vi "for testing.vi"() -> ()   [LabVIEW 2016] (continued)
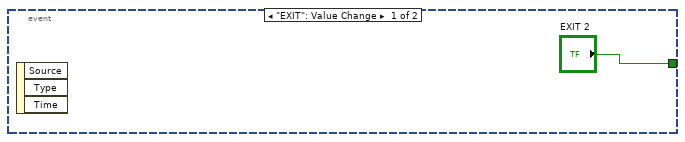
[diagram p2: hidden frame]
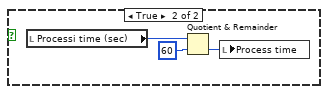
[diagram p3: hidden frame]
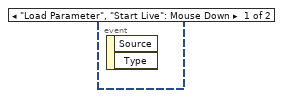
[diagram p4: hidden frame]
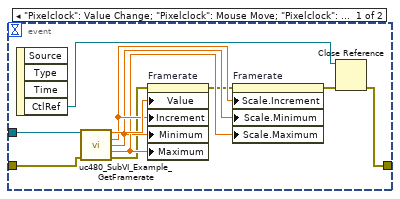
[diagram p5: hidden frame]
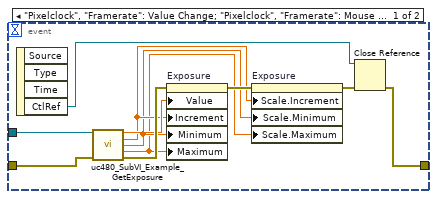
[diagram p6: hidden frame]
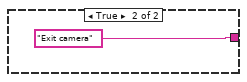
[diagram p7: hidden frame]
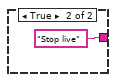
[diagram p8: hidden frame]
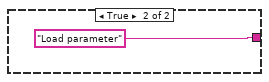
[diagram p9: hidden frame]
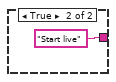
[diagram p10: hidden frame]
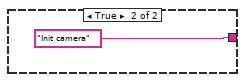
[diagram p11: hidden frame]
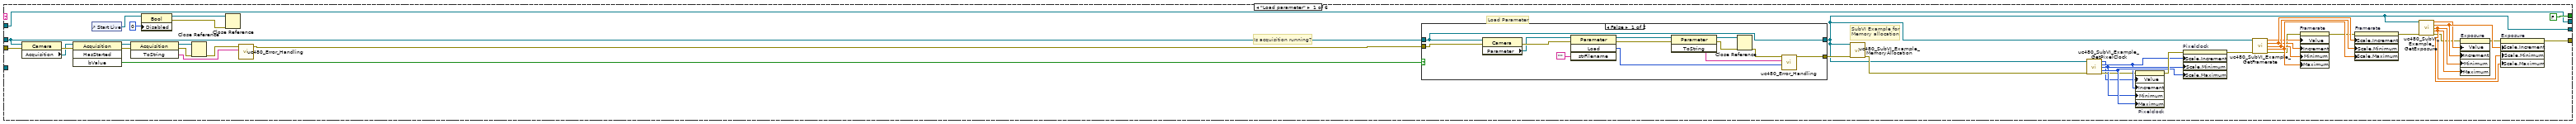
[diagram p12: hidden frame]
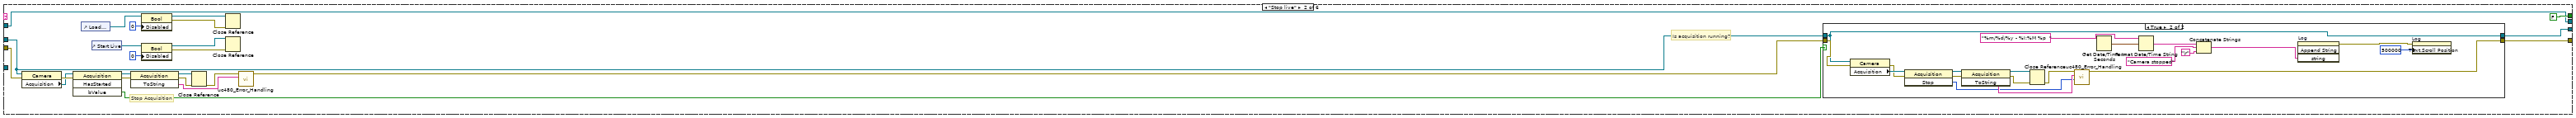
[diagram p14: hidden frame]
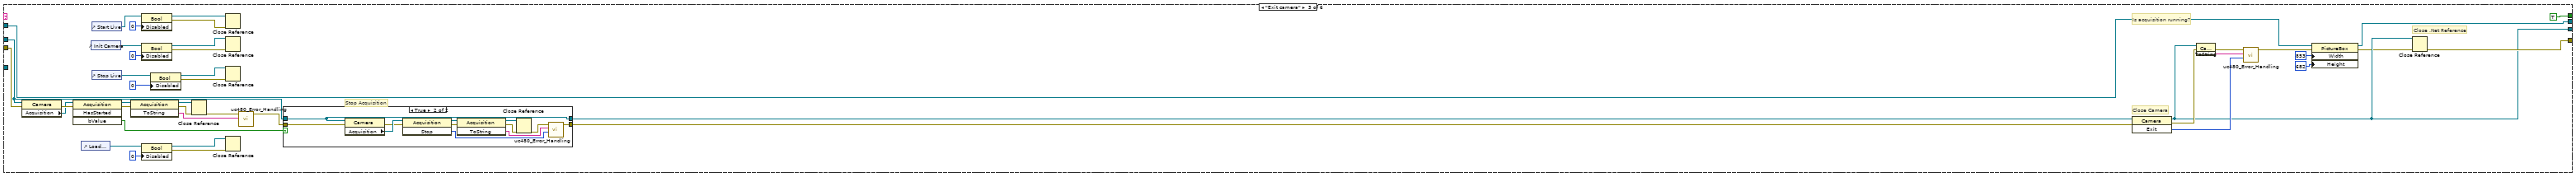
[diagram p16: hidden frame]
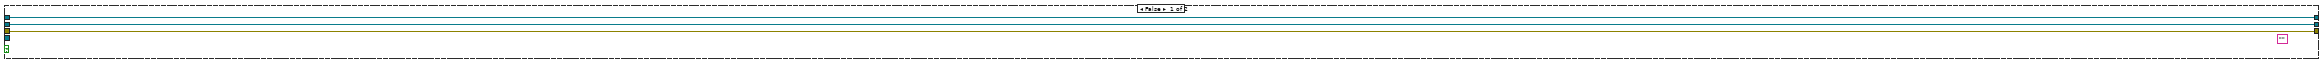
[diagram p18: hidden frame]
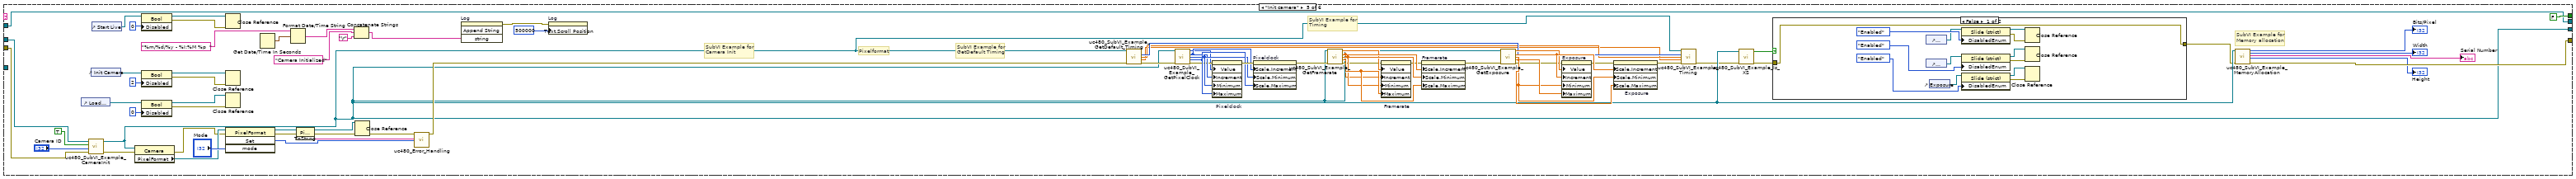
[diagram p20: hidden frame]
          }
          frame True {
            n522 = call "IR_Alignment_Diode.vi"("AD Action"=enum16{"AD Off", "AD On"}."AD On") -> ()  [unwired: 14 in, 1 out]
          }
        }
      }
      event "Open \nManual": Value Change {
        n523 = event-data() -> ()  [unwired: 1 in, 6 out]
        n524 = case shown="True" "Open \nManual" {
          tunnel: [_ "Opening Manual" ("StringOut")] -> w955
          frame False {
          }
          frame True {
            w962 = FALSE  # wait until completion? (T)
            n525 = control-ref of="This VI"() -> (w966:refnum<vi>)
            n526 = property class="VI"(reference=w966) -> ("Path"=w965:path)  [unwired: 1 in, 2 out]
            n527 = Strip Path(path=w965) -> (stripped path=w964:path)  [unwired: 1 out]
            n528 = Build Path(base path=w964, name or relative path="LAST_Software_Manual.PDF") -> (appended path=w958:path)
            n529 = Path To String(path=w958) -> (string=w959:string)
            n530 = Concatenate Strings("cmd  /c \"", w959, "\"" ("string")) -> (w956:string)
            n531 = call <vilib>:"System Exec.vi"("run minimized? (F)"=TRUE, "wait until completion? (T)"=w962, "command line"=w956) -> ()  [unwired: 5 in, 4 out]
          }
        }
      }
      event "Stages status": Value Change {
        w974 = "Ready"
        n532 = event-data() -> ()  [unwired: 1 in, 6 out]
        n533 = case shown="True" "Stages status" {
          tunnel: w983 -> [_ w996]
          tunnel: w982 -> [_ w995]
          tunnel: w981 -> [_ w994]
          tunnel: [w987 w993] -> w980
          tunnel: [w987 w991] -> w970
          tunnel: [w987 w992] -> w969
          frame False {
            w987 = ""
          }
          frame True {
            n534 = call <userlib>:"Open TCP-IP.vi"("IP address"=w996) -> ("error out"=w990:errorcluster, "Connection ID"=w997:T6)  [unwired: 8 in, 1 out]
            n535 = call <vilib>:"Simple Error Handler.vi"("error in (no error)"=w990) -> ("error?"=w988:bool, "error out"=w989:errorcluster)  [unwired: 4 in, 3 out]
            n536 = case shown="True" w988 {
              tunnel: w997 -> [w1018 _]
              tunnel: w989 -> [w1017 _]
              tunnel: w995 -> [w1010 _]
              tunnel: w994 -> [w1009 _]
              tunnel: [w1008 w1019] -> w993
              tunnel: [w1005 w1019] -> w992
              tunnel: [w1001 w1019] -> w991
              frame False {
                n537 = call "Get Stages Status.vi"("error in (no error)"=w1017, "Group Name (250 c max)"=w1010, "connection ID in"=w1018) -> ("error out"=w1014:errorcluster, "XPS error out"=w1013:errorcluster, "Group Status String"=w1005:string, "connection ID out"=w1016:T6)  [unwired: 4 in, 1 out]
                n538 = call "Get Stages Status.vi"("error in (no error)"=w1014, "XPS error in (no error)"=w1013, "Group Name (250 c max)"=w1009, "connection ID in"=w1016) -> ("error out"=w1011:errorcluster, "XPS error out"=w1007:errorcluster, "Group Status String"=w1001:string, "connection ID out"=w1012:T6)  [unwired: 3 in, 1 out]
                n539 = call <vilib>:"Simple Error Handler.vi"("error source (\" \")"="Stage status" ("error source (\" \")"), "error in (no error)"=w1007) -> ()  [unwired: 3 in, 5 out]
                n540 = Concatenate Strings("Axis 1 " ("string"), w1005) -> (w1004:string)
                n541 = call <userlib>:"Close TCP-IP.vi"("error in (no error)"=w1011, "connection ID in"=w1012) -> ("Error out"=w1006:errorcluster)  [unwired: 9 in]
                n542 = call <vilib>:"Simple Error Handler.vi"("error source (\" \")"="TCP close Stage status" ("error source (\" \")"), "error in (no error)"=w1006) -> ()  [unwired: 3 in, 5 out]
                n543 = Concatenate Strings("Axis 2 " ("string"), w1001) -> (w1002:string)
                n544 = Concatenate Strings(w1004, " - " ("string"), w1002) -> (w1008:string)
              }
              frame True {
                w1019 = ""
              }
            }
          }
        }
        n545 = String Subset(string=w969, offset (0)=0, length (rest)=5 ("length (rest)")) -> (substring=w973:string)
        n546 = String Subset(string=w970, offset (0)=0, length (rest)=5 ("length (rest)")) -> (substring=w975:string)
        n547 = Equal?(x=w974, y=w973) -> (x = y?=w971:bool)
        n548 = Equal?(x=w975, y=w974) -> (x = y?=w972:bool)
        n549 = And(x=w972, y=w971) -> (x .and. y?=w968:bool)
        n550 = case shown="True" w968 {
          frame False {
          }
          frame True {
            n551 = property on="Home Axes" class="Bool"("Visible"=TRUE) -> ()  [unwired: 2 in, 2 out]
            n552 = property on="Axes Manual Control" class="Bool (strict)"("Visible"=TRUE) -> ()  [unwired: 2 in, 2 out]
          }
        }
      }
      event "Save configuration": Value Change {
        n553 = event-data() -> ()  [unwired: 1 in, 6 out]
        n554 = case shown="True" "Save configuration" {
          frame False {
          }
          frame True {
            w1047 = "ROI Processing" ("section")
            n555 = control-ref of="This VI"() -> (w1053:refnum<vi>)
            n556 = property class="VI"(reference=w1053) -> ("Path"=w1052:path)  [unwired: 1 in, 2 out]
            n557 = Strip Path(path=w1052) -> (stripped path=w1051:path)  [unwired: 1 out]
            n558 = Build Path(base path=w1051, name or relative path="General_Configuration.ini") -> (appended path=w1049:path)
            n559 = local read "Heigth (µm)"() -> (w1033:i32)
            n560 = local read "Width (µm)"() -> (w1034:i32)
            n561 = local read "Pixel size"() -> (w1045:dbl)
            n562 = local read "X offset"() -> (w1032:i32)
            n563 = local read "Y offset"() -> (w1031:i32)
            n564 = local read "Height  step \ndivider"() -> (w1044:i32)
            n565 = call <vilib>:"Open Config Data.vi"("create file if necessary (T)"=FALSE, "configuration file path"=w1049) -> ("refnum"=w1021:T5)  [unwired: 7 in, 2 out]
            n566 = local read "Speed (µm/s)"() -> (w1035:i32)
            n567 = local read "Precision (%)"() -> (w1036:dbl)
            n568 = call-poly <vilib>:"Write Key.vi"("section"=w1047, "value"=w1045, "key"="Pixel Size", "refnum"=w1021) -> ("error out"=w1030:errorcluster)  [unwired: 5 in, 2 out]
            n569 = call-poly <vilib>:"Write Key.vi"("section"=w1047, "value"=w1044, "key"="Heigth step divider", "refnum"=w1021) -> ("error out"=w1029:errorcluster)  [unwired: 5 in, 2 out]
            n570 = call-poly <vilib>:"Write Key.vi"("section"=w1047, "value"=w1036, "key"="Precision (%)", "refnum"=w1021) -> ("error out"=w1028:errorcluster)  [unwired: 5 in, 2 out]
            n571 = call-poly <vilib>:"Write Key.vi"("section"=w1047, "value"=w1035, "key"="Sampling speed", "refnum"=w1021) -> ("error out"=w1027:errorcluster)  [unwired: 5 in, 2 out]
            n572 = call-poly <vilib>:"Write Key.vi"("section"=w1047, "value"=w1034, "key"="Width", "refnum"=w1021) -> ("error out"=w1026:errorcluster)  [unwired: 5 in, 2 out]
            n573 = call-poly <vilib>:"Write Key.vi"("section"=w1047, "value"=w1033, "key"="Height", "refnum"=w1021) -> ("error out"=w1025:errorcluster)  [unwired: 5 in, 2 out]
            n574 = call-poly <vilib>:"Write Key.vi"("section"=w1047, "value"=w1032, "key"="X offset", "refnum"=w1021) -> ("error out"=w1024:errorcluster)  [unwired: 5 in, 2 out]
            n575 = call-poly <vilib>:"Write Key.vi"("section"=w1047, "value"=w1031, "key"="Y offset", "refnum"=w1021) -> ("error out"=w1023:errorcluster)  [unwired: 5 in, 2 out]
            n576 = Merge Errors(w1030, w1029, w1028, w1027, w1026, w1025, w1024, w1023) -> (w1022:errorcluster)
            n577 = call <vilib>:"Close Config Data.vi"("error in (no error)"=w1022, "refnum"=w1021) -> ()  [unwired: 8 in, 2 out]
          }
        }
      }
      event "Axes Manual Control": Value Change {
        n578 = event-data() -> ()  [unwired: 1 in, 6 out]
        n579 = case shown="True" "Axes Manual Control" {
          tunnel: w1056 -> [_ w1068]
          tunnel: w1055 -> [_ w1067]
          tunnel: w1054 -> [_ w1066]
          frame False {
          }
          frame True {
            n580 = flat-sequence {
              tunnel: w1068 -> [w1078]
              tunnel: w1067 -> [w1077]
              tunnel: w1066 -> [w1076]
              tunnel: [w1078] -> w1065
              tunnel: [w1077] -> w1064
              tunnel: [w1076] -> w1063
              tunnel: [w1075] -> w1062
              tunnel: [w1074] -> w1061
              tunnel: [w1073] -> w1060
              tunnel: [w1072] -> w1059
              tunnel: w1065 -> [w1121]
              tunnel: w1064 -> [w1120]
              tunnel: w1063 -> [w1119]
              tunnel: w1062 -> [w1114]
              tunnel: w1061 -> [w1113]
              tunnel: w1060 -> [w1104]
              tunnel: w1059 -> [w1103]
              frame #0 {
                n581 = call <userlib>:"Open TCP-IP.vi"("IP address"=w1078) -> ("error out"=w1070:errorcluster, "Connection ID"=w1079:T6)  [unwired: 8 in, 1 out]
                n582 = call <vilib>:"Simple Error Handler.vi"("error in (no error)"=w1070) -> ("error?"=w1069:bool, "error out"=w1071:errorcluster)  [unwired: 4 in, 3 out]
                n583 = case shown="True" w1069 {
                  tunnel: w1079 -> [w1094 _]
                  tunnel: w1071 -> [w1093 _]
                  tunnel: w1077 -> [w1090 _]
                  tunnel: w1076 -> [w1089 _]
                  tunnel: [w1088 w1098] -> w1075
                  tunnel: [w1087 w1098] -> w1074
                  tunnel: [w1083 w1097] -> w1073
                  tunnel: [w1082 w1097] -> w1072
                  frame False {
                    n584 = call "Get Stages Status.vi"("error in (no error)"=w1093, "Group Name (250 c max)"=w1090, "connection ID in"=w1094) -> ("error out"=w1092:errorcluster, "XPS error out"=w1091:errorcluster, "Group Status String"=w1087:string, "connection ID out"=w1086:T6, "Status"=w1082:i32)  [unwired: 4 in]
                    n585 = call "Get Stages Status.vi"("error in (no error)"=w1092, "XPS error in (no error)"=w1091, "Group Name (250 c max)"=w1089, "connection ID in"=w1086) -> ("error out"=w1096:errorcluster, "XPS error out"=w1085:errorcluster, "Group Status String"=w1088:string, "connection ID out"=w1095:T6, "Status"=w1083:i32)  [unwired: 3 in]
                    n586 = call <vilib>:"Simple Error Handler.vi"("error source (\" \")"="Axis manual control check" ("error source (\" \")"), "error in (no error)"=w1085) -> ()  [unwired: 3 in, 5 out]
                    n587 = call <userlib>:"Close TCP-IP.vi"("error in (no error)"=w1096, "connection ID in"=w1095) -> ("Error out"=w1084:errorcluster)  [unwired: 9 in]
                    n588 = call <vilib>:"Simple Error Handler.vi"("error source (\" \")"="TCP close Axis manual control check" ("error source (\" \")"), "error in (no error)"=w1084) -> ()  [unwired: 3 in, 5 out]
                  }
                  frame True {
                    w1097 = 0
                    w1098 = ""
                  }
                }
              }
              frame #1 {
                w1107 = 47 ("y")
                w1108 = "Ready"
                n589 = String Subset(string=w1113, offset (0)=0, length (rest)=5 ("length (rest)")) -> (substring=w1110:string)
                n590 = String Subset(string=w1114, offset (0)=0, length (rest)=5 ("length (rest)")) -> (substring=w1109:string)
                n591 = Equal?(x=w1110, y=w1108) -> (x = y?=w1111:bool)
                n592 = Equal?(x=w1108, y=w1109) -> (x = y?=w1112:bool)
                n593 = Equal?(x=w1107, y=w1103) -> (x = y?=w1105:bool)
                n594 = Equal?(x=w1104, y=w1107) -> (x = y?=w1106:bool)
                n595 = And(x=w1106, y=w1105) -> (x .and. y?=w1100:bool)
                n596 = And(x=w1111, y=w1112) -> (x .and. y?=w1101:bool)
                n597 = Not(x=w1100) -> (.not. x?=w1099:bool)
                n598 = And(x=w1101, y=w1099) -> (x .and. y?=w1102:bool)
                n599 = case shown="True" w1102 {
                  tunnel: w1121 -> [_ w1127]
                  tunnel: w1120 -> [_ w1126]
                  tunnel: w1119 -> [_ w1125]
                  tunnel: w1099 -> [w1122 _]
                  frame False {
                    n600 = case shown="False" w1122 {
                      frame False {
                        n601 = One Button Dialog(message="One or more axis already in jogging position") -> ()  [unwired: 1 in, 1 out]
                      }
                      frame True {
                        n602 = One Button Dialog(message="Axes are not ready") -> ()  [unwired: 1 in, 1 out]
                      }
                    }
                  }
                  frame True {
                    n603 = call "XPS_LTA_HS_Jogger.vi"("Axis 2"=w1125, "Axis 1"=w1126, "Controller Address"=w1127) -> ()  [unwired: 8 in]
                  }
                }
              }
            }
          }
        }
      }
      event "Home Axes": Value Change {
        n604 = event-data() -> ()  [unwired: 1 in, 6 out]
        n605 = flat-sequence {
          tunnel: w1134 -> [w1140]
          tunnel: w1135 -> [w1141]
          tunnel: w1136 -> [w1142]
          tunnel: "Home Axes" -> [w1143]
          tunnel: [w1143] -> w1132
          tunnel: [w1142] -> w1131
          tunnel: [w1141] -> w1130
          tunnel: [w1140] -> w1129
          tunnel: [w1139] -> w1128
          tunnel: [w1147] -> w1133
          tunnel: w1132 -> [w1145]
          tunnel: w1131 -> [w1150]
          tunnel: w1130 -> [w1148]
          tunnel: w1129 -> [w1149]
          tunnel: w1128 -> [w1146]
          tunnel: [w1229] -> w1137
          tunnel: w1133 -> [w1228]
          frame #0 {
            n606 = call "Display Message to User"() -> ("OK"=w1139:bool)  [unwired: 10 in, 1 out]
          }
          frame #1 {
            n607 = And(x=w1145, y=w1146) -> (x .and. y?=w1144:bool)
            n608 = case shown="True" w1144 {
              tunnel: w1150 -> [_ w1166]
              tunnel: w1148 -> [_ w1167]
              tunnel: w1149 -> [_ w1164]
              tunnel: w1148 -> [_ w1165]
              tunnel: [FALSE w1157] -> w1147
              frame False {
              }
              frame True {
                w1163 = 47 ("y")
                w1179 = "Ready"
                n609 = call <userlib>:"Open TCP-IP.vi"("IP address"=w1166) -> ("error out"=w1152:errorcluster, "Connection ID"=w1170:T6)  [unwired: 8 in, 1 out]
                n610 = call <vilib>:"Simple Error Handler.vi"("error in (no error)"=w1152) -> ("error?"=w1154:bool, "error out"=w1153:errorcluster)  [unwired: 4 in, 3 out]
                n611 = case shown="True" w1154 {
                  tunnel: w1153 -> [w1193 _]
                  tunnel: w1170 -> [w1192 _]
                  tunnel: [w1189 w1198] -> w1169
                  tunnel: [w1188 w1198] -> w1168
                  tunnel: w1167 -> [w1187 _]
                  tunnel: w1164 -> [w1186 _]
                  tunnel: [w1183 w1197] -> w1162
                  tunnel: [w1182 w1197] -> w1161
                  frame False {
                    n612 = call "Get Stages Status.vi"("error in (no error)"=w1193, "Group Name (250 c max)"=w1187, "connection ID in"=w1192) -> ("error out"=w1194:errorcluster, "XPS error out"=w1195:errorcluster, "Group Status String"=w1189:string, "connection ID out"=w1196:T6, "Status"=w1182:i32)  [unwired: 4 in]
                    n613 = call "Get Stages Status.vi"("error in (no error)"=w1194, "XPS error in (no error)"=w1195, "Group Name (250 c max)"=w1186, "connection ID in"=w1196) -> ("error out"=w1190:errorcluster, "XPS error out"=w1185:errorcluster, "Group Status String"=w1188:string, "connection ID out"=w1191:T6, "Status"=w1183:i32)  [unwired: 3 in]
                    n614 = call <vilib>:"Simple Error Handler.vi"("error source (\" \")"="home axis check" ("error source (\" \")"), "error in (no error)"=w1185) -> ()  [unwired: 3 in, 5 out]
                    n615 = call <userlib>:"Close TCP-IP.vi"("error in (no error)"=w1190, "connection ID in"=w1191) -> ("Error out"=w1184:errorcluster)  [unwired: 9 in]
                    n616 = call <vilib>:"Simple Error Handler.vi"("error source (\" \")"="TCP close home axis check" ("error source (\" \")"), "error in (no error)"=w1184) -> ()  [unwired: 3 in, 5 out]
                  }
                  frame True {
                    w1197 = 0
                    w1198 = ""
                  }
                }
                n617 = Equal?(x=w1163, y=w1161) -> (x = y?=w1160:bool)
                n618 = Equal?(x=w1162, y=w1163) -> (x = y?=w1159:bool)
                n619 = String Subset(string=w1169, offset (0)=0, length (rest)=5 ("length (rest)")) -> (substring=w1177:string)
                n620 = String Subset(string=w1168, offset (0)=0, length (rest)=5 ("length (rest)")) -> (substring=w1178:string)
                n621 = Equal?(x=w1177, y=w1179) -> (x = y?=w1176:bool)
                n622 = Equal?(x=w1179, y=w1178) -> (x = y?=w1175:bool)
                n623 = And(x=w1159, y=w1160) -> (x .and. y?=w1155:bool)
                n624 = Not(x=w1155) -> (.not. x?=w1156:bool)
                n625 = And(x=w1176, y=w1175) -> (x .and. y?=w1158:bool)
                n626 = And(x=w1158, y=w1156) -> (x .and. y?=w1157:bool)
                n627 = case shown="True" w1157 {
                  tunnel: w1166 -> [_ w1208]
                  tunnel: w1165 -> [_ w1207]
                  tunnel: w1164 -> [_ w1206]
                  tunnel: w1155 -> [w1199 _]
                  frame False {
                    n628 = case shown="True" w1199 {
                      frame False {
                        n629 = One Button Dialog(message="Axes are not ready") -> ()  [unwired: 1 in, 1 out]
                      }
                      frame True {
                        n630 = One Button Dialog(message="One or more axis are in jogging mode") -> ()  [unwired: 1 in, 1 out]
                      }
                    }
                  }
                  frame True {
                    n631 = call <userlib>:"Open TCP-IP.vi"("IP address"=w1208) -> ("error out"=w1224:errorcluster, "Connection ID"=w1225:T6)  [unwired: 8 in, 1 out]
                    n632 = call <userlib>:"Group Kill.vi"("error in (no error)"=w1224, "Group Name (250 c max)"=w1207, "connection ID in"=w1225) -> ("error out"=w1222:errorcluster, "XPS error out"=w1223:errorcluster, "connection ID out"=w1219:T6)  [unwired: 6 in]
                    n633 = call <userlib>:"Group Initialize.vi"("error in (no error)"=w1222, "XPS error in (no error)"=w1223, "Group Name (250 c max)"=w1207, "connection ID in"=w1219) -> ("error out"=w1220:errorcluster, "XPS error out"=w1221:errorcluster, "connection ID out"=w1218:T6)  [unwired: 5 in]
                    n634 = call <userlib>:"Group Home Search.vi"("error in (no error)"=w1220, "XPS error in (no error)"=w1221, "Group Name (250 c max)"=w1207, "connection ID in"=w1218) -> ("error out"=w1209:errorcluster, "XPS error out"=w1210:errorcluster, "connection ID out"=w1217:T6)  [unwired: 5 in]
                    n635 = call <userlib>:"Group Kill.vi"("error in (no error)"=w1209, "XPS error in (no error)"=w1210, "Group Name (250 c max)"=w1206, "connection ID in"=w1217) -> ("error out"=w1211:errorcluster, "XPS error out"=w1212:errorcluster, "connection ID out"=w1216:T6)  [unwired: 5 in]
                    n636 = call <userlib>:"Group Initialize.vi"("error in (no error)"=w1211, "XPS error in (no error)"=w1212, "Group Name (250 c max)"=w1206, "connection ID in"=w1216) -> ("error out"=w1213:errorcluster, "XPS error out"=w1214:errorcluster, "connection ID out"=w1215:T6)  [unwired: 5 in]
                    n637 = call <userlib>:"Group Home Search.vi"("error in (no error)"=w1213, "XPS error in (no error)"=w1214, "Group Name (250 c max)"=w1206, "connection ID in"=w1215) -> ("error out"=w1226:errorcluster, "XPS error out"=w1205:errorcluster, "connection ID out"=w1227:T6)  [unwired: 5 in]
                    n638 = call <vilib>:"Simple Error Handler.vi"("error source (\" \")"="home axis " ("error source (\" \")"), "error in (no error)"=w1205) -> ()  [unwired: 3 in, 5 out]
                    n639 = call <userlib>:"Close TCP-IP.vi"("error in (no error)"=w1226, "connection ID in"=w1227) -> ("Error out"=w1204:errorcluster)  [unwired: 9 in]
                    n640 = call <vilib>:"Simple Error Handler.vi"("error source (\" \")"="TCP close home axis " ("error source (\" \")"), "error in (no error)"=w1204) -> ()  [unwired: 3 in, 5 out]
                  }
                }
              }
            }
          }
          frame #2 {
            n641 = case shown="True" w1228 {
              tunnel: ["" ("StringOut") "Axes have been moved to home position" ("StringOut")] -> w1229
              frame False {
              }
              frame True {
              }
            }
          }
        }
      }
      event "Transparency": Value Change {
        n642 = event-data() -> ()  [unwired: 1 in, 6 out]
        n643 = control-ref of="This VI"() -> (w1233:refnum<vi>)
        n644 = property class="VI"(reference=w1233, "FP:Transparency"="Transparency") -> ()  [unwired: 1 in, 2 out]
      }
      event "Capture": Value Change {
        w1244 = 47 ("y")
        w1260 = "Ready"
        n645 = event-data() -> ()  [unwired: 1 in, 6 out]
        n646 = call <userlib>:"Open TCP-IP.vi"("IP address"=w1248) -> ("error out"=w1236:errorcluster, "Connection ID"=w1251:T6)  [unwired: 8 in, 1 out]
        n647 = call <vilib>:"Simple Error Handler.vi"("error in (no error)"=w1236) -> ("error?"=w1234:bool, "error out"=w1235:errorcluster)  [unwired: 4 in, 3 out]
        n648 = case shown="True" w1234 {
          tunnel: w1235 -> [w1274 _]
          tunnel: w1251 -> [w1273 _]
          tunnel: [w1270 w1278] -> w1250
          tunnel: [w1269 w1278] -> w1249
          tunnel: w1247 -> [w1268 _]
          tunnel: w1246 -> [w1267 _]
          tunnel: [w1265 w1279] -> w1245
          tunnel: [w1264 w1279] -> w1243
          frame False {
            n649 = call "Get Stages Status.vi"("error in (no error)"=w1274, "Group Name (250 c max)"=w1268, "connection ID in"=w1273) -> ("error out"=w1275:errorcluster, "XPS error out"=w1276:errorcluster, "Group Status String"=w1270:string, "connection ID out"=w1277:T6, "Status"=w1264:i32)  [unwired: 4 in]
            n650 = call "Get Stages Status.vi"("error in (no error)"=w1275, "XPS error in (no error)"=w1276, "Group Name (250 c max)"=w1267, "connection ID in"=w1277) -> ("error out"=w1271:errorcluster, "XPS error out"=w1266:errorcluster, "Group Status String"=w1269:string, "connection ID out"=w1272:T6, "Status"=w1265:i32)  [unwired: 3 in]
            n651 = call <vilib>:"Simple Error Handler.vi"("error source (\" \")"="Capture check" ("error source (\" \")"), "error in (no error)"=w1266) -> ()  [unwired: 3 in, 5 out]
            n652 = call <userlib>:"Close TCP-IP.vi"("error in (no error)"=w1271, "connection ID in"=w1272) -> ("Error out"=w1262:errorcluster)  [unwired: 9 in]
            n653 = call <vilib>:"Simple Error Handler.vi"("error in (no error)"=w1262) -> ()  [unwired: 4 in, 5 out]
          }
          frame True {
            w1279 = 0
            w1278 = ""
          }
        }
        n654 = Equal?(x=w1244, y=w1243) -> (x = y?=w1241:bool)
        n655 = Equal?(x=w1245, y=w1244) -> (x = y?=w1242:bool)
        n656 = String Subset(string=w1250, offset (0)=0, length (rest)=5 ("length (rest)")) -> (substring=w1258:string)
        n657 = String Subset(string=w1249, offset (0)=0, length (rest)=5 ("length (rest)")) -> (substring=w1259:string)
        n658 = Equal?(x=w1258, y=w1260) -> (x = y?=w1257:bool)
        n659 = Equal?(x=w1260, y=w1259) -> (x = y?=w1256:bool)
        n660 = And(x=w1242, y=w1241) -> (x .and. y?=w1238:bool)
        n661 = And(x=w1257, y=w1256) -> (x .and. y?=w1240:bool)
        n662 = Not(x=w1238) -> (.not. x?=w1237:bool)
        n663 = And(x=w1240, y=w1237) -> (x .and. y?=w1239:bool)
        n664 = case shown="True" w1239 {
          tunnel: ["" w1287] -> w1261
          tunnel: w1248 -> [_ w1286]
          tunnel: w1246 -> [_ w1285]
          tunnel: w1247 -> [_ w1284]
          tunnel: w1238 -> [w1280 _]
          frame False {
            n665 = case shown="True" w1280 {
              frame False {
                n666 = One Button Dialog(message="Axes are not ready") -> ()  [unwired: 1 in, 1 out]
              }
              frame True {
                n667 = One Button Dialog(message="One or more axis are in jogging mode") -> ()  [unwired: 1 in, 1 out]
              }
            }
          }
          frame True {
            n668 = flat-sequence {
              tunnel: [w1308] -> w1299
              tunnel: [w1307] -> w1298
              tunnel: [w1306] -> w1297
              tunnel: [w1305] -> w1296
              tunnel: [w1304] -> w1295
              tunnel: [w1303] -> w1294
              tunnel: [w1302] -> w1293
              tunnel: w1286 -> [w1302]
              tunnel: w1285 -> [w1301]
              tunnel: w1284 -> [w1300]
              tunnel: w1299 -> [w1328]
              tunnel: w1298 -> [w1319]
              tunnel: w1297 -> [w1320]
              tunnel: w1296 -> [w1326]
              tunnel: w1295 -> [w1325]
              tunnel: [w1318] -> w1292
              tunnel: w1294 -> [w1318]
              tunnel: [w1317] -> w1291
              tunnel: w1293 -> [w1317]
              tunnel: [w1330] -> w1290
              tunnel: w1292 -> [w1330]
              tunnel: [w1329] -> w1289
              tunnel: w1291 -> [w1329]
              tunnel: w1290 -> [w1335]
              tunnel: w1289 -> [w1340]
              tunnel: [w1334] -> w1288
              tunnel: [w1350] -> w1287
              tunnel: w1288 -> [w1347]
              frame #0 {
                w1313 = ".Pos"
                n669 = local read "Axis Initial Parameters"() -> (w1303:T2)
                n670 = Concatenate Strings(w1300, w1313) -> (w1307:string)
                n671 = call <userlib>:"Open TCP-IP.vi"("IP address"=w1302) -> ("error out"=w1309:errorcluster, "Connection ID"=w1314:T6)  [unwired: 5 in, 4 out]
                n672 = call <userlib>:"Positioner SGamma Parameters Set.vi"("SGamma Parameters"=w1303, "error in (no error)"=w1309, "Positioner Name (250 c max)"=w1307, "connection ID in"=w1314) -> ("error out"=w1310:errorcluster, "XPS error out"=w1311:errorcluster, "connection ID out"=w1312:T6)  [unwired: 5 in]
                n673 = Concatenate Strings(w1301, w1313) -> (w1306:string)
                n674 = call <userlib>:"Positioner SGamma Parameters Set.vi"("SGamma Parameters"=w1303, "error in (no error)"=w1310, "XPS error in (no error)"=w1311, "Positioner Name (250 c max)"=w1306, "connection ID in"=w1312) -> ("error out"=w1305:errorcluster, "XPS error out"=w1304:errorcluster, "connection ID out"=w1308:T6)  [unwired: 4 in]
              }
              frame #1 {
                n675 = local read "Axis 2 Offset"() -> (w1316:dbl)
                n676 = local read "Axis 1 Offset"() -> (w1315:dbl)
                n677 = call <userlib>:"Single Axis Group Move Relative.vi"("Target Displacement (units)"=w1316, "error in (no error)"=w1326, "XPS error in (no error)"=w1325, "SingleAxis Group  Name (250 c max)"=w1319, "connection ID in"=w1328) -> ("error out"=w1323:errorcluster, "XPS error out"=w1324:errorcluster, "connection ID out"=w1327:T6)  [unwired: 4 in]
                n678 = call <userlib>:"Single Axis Group Move Relative.vi"("Target Displacement (units)"=w1315, "error in (no error)"=w1323, "XPS error in (no error)"=w1324, "SingleAxis Group  Name (250 c max)"=w1320, "connection ID in"=w1327) -> ("error out"=w1321:errorcluster, "connection ID out"=w1322:T6)  [unwired: 4 in, 1 out]
                n679 = call <userlib>:"Close TCP-IP.vi"("error in (no error)"=w1321, "connection ID in"=w1322) -> ()  [unwired: 9 in, 1 out]
              }
              frame #2 {
                n680 = Wait (ms)(milliseconds to wait=u32 1000) -> ()  [unwired: 1 out]
              }
              frame #3 {
                n681 = local read "Speed (µm/s)"() -> (w1339:i32)
                n682 = local read "Processi time (sec)"() -> (w1333:i32)
                n683 = local read "Laser on/off array"() -> (w1344:bool[][])
                n684 = local read "Alignment \ndiode"() -> (w1343:bool)
                n685 = local read "Commands array"() -> (w1345:string[][])
                n686 = Divide(x=w1339, y=1000) -> (x/y=w1336:dbl)
                n687 = call "IR_OPO_Capture_V2.vi"("Commands array"=w1345, "Laser on/off array"=w1344, "AD status"=w1343, "XPS_Address"=w1340, "laser array index"=0, "OPO on?"=TRUE, "Process time"=w1333, "Axis Speed"=w1336, "stop"=FALSE ("STOP CAPTURE"), "Axis Initial Parameters"=w1335, "Acceleration (units/seconds²)"="Acceleration \n(mm/s²)") -> ("Elapsed time"=w1334:dbl)  [unwired: 4 in]
              }
              frame #4 {
                n688 = Number To Decimal String(number=w1347) -> (decimal integer string=w1346:string)  [unwired: 1 in]
                n689 = Concatenate Strings("Capture completed in " ("StringOut"), w1346, " seconds" ("string")) -> (w1350:string)
              }
            }
          }
        }
      }
    }
    n690 = Get Date/Time In Seconds() -> (seconds since 1Jan1904=w842:timestamp)
    n691 = Format Date/Time String(time format string (%c)="%m/%d/%y - %I:%M %p  ", seconds (now)=w842) -> (date/time string=w841:string)  [unwired: 1 in]
    n692 = Empty String/Path?(string/path=w838) -> (empty?=w840:bool)
    n693 = Concatenate Strings(w841, w838, "\r") -> (w839:string)
    n694 = case shown="False" w840 {
      tunnel: w839 -> [w848 _]
      frame False {
        n695 = invoke on="Log" class="Str" method="Append String"("string"=w848) -> (error out=w847:errorcluster)  [unwired: 3 in, 3 out]
        n696 = property on="Log" class="Str"(error in=w847, "Text.Scroll Position"=u32 500000) -> ()  [unwired: 1 in, 2 out]
      }
      frame True {
      }
    }
  }
  n697 = while "Processing Time Unit" {
    stop <- w1351 stop-if-true
    n698 = event shown="[1] \"Processing time unit\", \"Processi time (sec)\": Value Change" {
      selector: _ -> [_ _]
      dyn-events: _ -> [_ _]
      timeout: _ -> [_ _]
      tunnel: ["EXIT 2" _] -> w1351
      event "EXIT": Value Change {
        n699 = event-data() -> ()  [unwired: 1 in, 3 out]
      }
      event "Processing time unit", "Processi time (sec)": Value Change {
        n700 = event-data() -> ()  [unwired: 1 in, 4 out]
        n701 = local read "Processing time unit"() -> (w1355:string)
        n702 = Equal?(x=w1355, y="min") -> (x = y?=w1353:bool)
        n703 = case shown="False" w1353 {
          frame False {
            n704 = local read "Processi time (sec)"() -> (w1356:i32)
            n705 = local write "Process time"(w1356) -> ()
          }
          frame True {
            n706 = local read "Processi time (sec)"() -> (w1358:i32)
            n707 = Quotient & Remainder(x=w1358, y=60) -> (floor(x/y)=w1357:i32)  [unwired: 1 out]
            n708 = local write "Process time"(w1357) -> ()
          }
        }
      }
    }
  }
  n709 = control-ref of="Init Camera"() -> (w25:refnum<vi>)
  n710 = control-ref of="Stop Live"() -> (w18:refnum<vi>)
  n711 = property class="Bool"(reference=w18, "Disabled"=u8 2 ("Deaktiviert")) -> (reference out=w9:refnum<vi>, error out=w8:errorcluster)  [unwired: 1 in]
  n712 = property class="Bool"(reference=w25, "Disabled"=u8 0 ("Deaktiviert")) -> (reference out=w13:refnum<vi>, error out=w12:errorcluster)  [unwired: 1 in]
  n713 = Close Reference(reference=w9, error in (no error)=w8) -> ()  [unwired: 1 out]
  n714 = Close Reference(reference=w13, error in (no error)=w12) -> ()  [unwired: 1 out]
  n715 = control-ref of="Load Parameter"() -> (w19:refnum<vi>)
  n716 = control-ref of="Start Live"() -> (w22:refnum<vi>)
  n717 = property class="Bool"(reference=w22, "Disabled"=u8 2 ("Deaktiviert")) -> (reference out=w11:refnum<vi>, error out=w10:errorcluster)  [unwired: 1 in]
  n718 = property class="Bool"(reference=w19, "Disabled"=u8 2 ("Deaktiviert")) -> (reference out=w7:refnum<vi>, error out=w6:errorcluster)  [unwired: 1 in]
  n719 = Close Reference(reference=w11, error in (no error)=w10) -> ()  [unwired: 1 out]
  n720 = Close Reference(reference=w7, error in (no error)=w6) -> ()  [unwired: 1 out]
